vi "UHR-Fleezers Control (host) - 12.4.vi"() -> ()   [LabVIEW 2012] (continued)
  T20 = enum16{"empty", "write", "read oldest (queue)", "read newest (stack)", "read all"}
  T21 = cluster{"New Image":T2, "New Image":T2, "New Image":T2, "New Image":T2, "New Image":T2}
  T22 = typedef "XDNodeRunTimeDep.lvlib/timing_clust.ctl" = cluster{"Expected End [f-1]":u64, "Actual End [f-1]":u64, "Finished Late? [f-1]":bool, "Expected End [i-1]":u64, "Actual End [i-1]":u64, "Finished Late? [i-1]":bool, "Expected Start [i]":u64, "Actual Start [i]":u64, "Expected Start [f]":u64, "Actual Start [f]":u64, "Source Name":string, "Structure Name":string, "Period":i64, "Deadline":i64, "Offset":i64, "Start":i64, "Priority":i32, "Timeout":i32, "Mode":T23, "Wakeup Reason":T24, "Error":errorcluster, "Source Type":string, "Secondary Source Type":string, "Global End Time":u64, "Global Start Time":u64, "Frame Duration":u64, "Iteration Duration":u64, "Assigned CPU":i32, "I/O Scan Engine Mode":u32}
  T23 = typedef "XDNodeRunTimeDep.lvlib/nitl_modes.ctl" = enum32{"No Change", "Process missed periods, maintain original phase", "Discard missed periods, maintain original phase", "Process missed periods, ignore original phase", "Discard missed periods, ignore original phase"}
  T24 = typedef "XDNodeRunTimeDep.lvlib/wakeup.ctl" = enum32{"Normal", "Aborted", "Asynchronous wakeup", "Timing source error", "Timed loop error", "Timeout"}
  T25 = enum32{"Status", "Sample Stage", "Syringe Pump", "Trap Control (RF)", "APD Counting", "Fluorescence Laser Control", "Trap AI", "Video", "FPGA"}
  T26 = enum16{"big-endian, network order", "native, host order", "little-endian"}
  T27 = enum16{"open", "replace", "create", "open or create", "replace or create", "replace or create with confirmation"}
  T28 = cluster{"Scan Range AOD (nm) 2":dbl, "Step Size AOD (nm) 2":dbl, "Scan Speed AOD (nm/s) 2":dbl, "Number of scans (AOD) 2":u16, "Label":string}
  T29 = cluster{"[0]":dbl, "[1]":dbl, "[2]":dbl, "[3]":dbl, "[4]":dbl, "[5]":dbl}
  T30 = cluster{"Diameter (mm)":dbl, "Units":dbl, "Volume":dbl, "Rate":dbl}
  T31 = cluster{"Left":i32, "Top":i32, "Width":u32, "Height":u32}
  T32 = cluster{cluster{"Left":i32, "Top":i32, "Width":u32, "Height":u32}}[]
  T33 = enum32{"Normal Display", "Dual Display (APD)", "FFT", "High Res Display"}
  T34 = cluster{"Origin Pixel":cluster{"X":sgl, "Y":sgl}, "Angle Relative to Horizontal (deg)":sgl, "Axis Reference":u32}
  T35 = typedef "Simple Grid Descriptor" = cluster{"X Step":sgl, "Y Step":sgl, "Unit":T36}
  T36 = typedef "Image Unit" = enum32{"Undefined", "Angström", "Micrometer", "Millimeter", "Centimeter", "Meter", "Kilometer", "Microinch", "Inch", "Feet", "Nautical miles", "Standard miles", "Steps"}
  T37 = cluster{"averaging mode":u16, "weighting mode":u16, "number of averages":u32}
  T38 = cluster{"dB On (F)":bool, "unwrap phase (F)":bool, "convert to degree (F)":bool}
  T39 = cluster{string, string, string, string, string, string, string, string}
  T40 = cluster{string, string, string, string, string, string, string, string, string, string, string, string}
  T41 = cluster{string, string, string, string, string, string, string, string, string, string, string, string, string}
  T42 = cluster{string, string, string, string, string, string, string, string, string, string, string, string, string, string}
  T43 = cluster{"BD 1 Frequency 1 (MHz)":dbl, "BD 1 Frequency 2 (MHz)":dbl}
  T44 = cluster{"f0":dbl, "df":dbl, "magnitude":dbl[]}[][]
  T45 = enum32{"setting", "request", "request control", "info", "statistics", "system settings", "I/O sub system", "HRT control", "camera descriptions", "device specific data", "event sub system settings", "event sub system results", "image memory manager"}
  T46 = typedef "AviRefnum.ctl" = refnum<k1>
  T47 = typedef "imagedata.ctl" = cluster{"image type":i32, "image depth":i32, "image":u8[], "mask":u8[], "colors":u32[], "Rectangle":cluster{"left":i16, "top":i16, "right":i16, "bottom":i16}}
diagram:
  w3 = u16 10 items=["1.0"=10, "1.5"=15, "2.0"=20] ("stop bits (10: 1 bit)")
  w74 = u16 20 items=["1.0"=10, "1.5"=15, "2.0"=20] ("stop bits (10: 1 bit)")
  w77 = u16 20 items=["1.0"=10, "1.5"=15, "2.0"=20] ("stop bits (10: 1 bit)")
  w103 = u16 20 items=["1.0"=10, "1.5"=15, "2.0"=20] ("stop bits (10: 1 bit)")
  w9 = T17 2 items=["Grayscale (U8)", "Grayscale (I16)", "Grayscale (SGL)", "Complex (CSG)", "RGB (U32)", "HSL (U32)", "RGB (U64)", "Grayscale (U16)"] ("Image Type")
  w233 = 10.0 ("y")
  w232 = 32767.0 ("y")
  w248 = 6.0  # clock mult.
  w249 = 49152000.0  # TCXO frequ.
  # "What are these?"
  # "I don't think you need to do this.\nEverytime you want to adjust phase you always set this anyway.\nSince we removed the separate +/- controls.\n\nHaven't added for added fl lasers.  Should remove this code."
  # "Bottom 1 Harvard"
  # "Top 3 Harvard"
  # "Center Harvard"
  # "Bottom 1 Harvard"
  # "Top 3 Harvard"
  # "Center Harvard"
  n1 = Build Array("DIO count 1 (ticks)", "DIO count 2 (ticks)", "DIO count 3 (ticks)") -> (w154:u16[])
  n2 = xnode "Open FPGA VI Reference"("resource name"=T18 "750kHzDAQ") -> ("FPGA VI Reference Out"=w257:T19, "error out"=w256:errorcluster)  [unwired: 1 in]
  n3 = local read "AO1"() -> (w227:dbl)
  n4 = local read "AO2"() -> (w226:dbl)
  n5 = local read "Scan Increment (MHz)"() -> (w244:dbl)
  n6 = local read "Continuous MCL Scanning"() -> (w214:bool)
  n7 = local read "Fast Scan Dir"() -> (w213:bool)
  n8 = xnode "Invoke Method"("FPGA VI Reference In"=w257, "error in"=w256) -> ("FPGA VI Reference Out"=w13:T19, "error out"=w173:errorcluster)
  n9 = local read "Number of scans (MCL)"() -> (w215:u64)
  n10 = Multiply(x=w227, y=w232) -> (x*y=w229:dbl)
  n11 = Multiply(x=w226, y=w232) -> (x*y=w231:dbl)
  n12 = Divide(x=w229, y=w233) -> (x/y=w228:dbl)
  n13 = Divide(x=w231, y=w233) -> (x/y=w230:dbl)
  n14 = To Word Integer(number=w228) -> (16bit integer=w225:i16)
  n15 = To Word Integer(number=w230) -> (16bit integer=w224:i16)
  n16 = Not(x=w213) -> (.not. x?=w208:bool)
  n17 = local read "Cycles/step (MCL)"() -> (w216:u64)
  n18 = Multiply(x=w244, y=1000.0) -> (x*y=w251:dbl)
  n19 = local read "Scan steps (MCL)"() -> (w217:u64)
  n20 = local read "Desired Scan Incr (V)"() -> (w219:dbl)
  n21 = Scale By Power Of 2(n=48, x=w251) -> (x*2^n=w252:dbl)
  n22 = Unbundle By Name(cluster{"output high":i16, "output low":i16} {"output high"=3000, "output low"=0} ("FB output range 1")) -> ("output high"=w55:i16, "output low"=w54:i16)
  n23 = Multiply(x=w249, y=w248) -> (x*y=w247:dbl)
  n24 = Divide(x=w252, y=w247) -> (x/y=w246:dbl)
  n25 = local read "Setpoints (V)"() -> (w263:cluster{"Set 1":dbl, "Set 2":dbl})
  n26 = To Quad Integer(1:w246) -> (0:w243:i64)
  n27 = Divide(x=40000000.0, y="AI Count (ticks)") -> (x/y=w204:dbl)
  n28 = Multiply(x=w219, y=32767.0) -> (x*y=w221:dbl)
  n29 = local read "Trap Intensity PID Gains"() -> (w258:T9)
  n30 = local write "Trap Pos FIFO Timeout"(u16 0 ("Trap Pos FIFO Timeout")) -> ()
  n31 = local read "Number Interlace Sets"() -> (w147:u8)
  n32 = Split 1D Array(array=w154, index=w147) -> (first subarray=w156:u16[])  [unwired: 1 out]
  n33 = Add Array Elements(numeric array=w156) -> (sum=w155:u16)
  n34 = local read "# Samples/channel"() -> (w236:u32)
  n35 = local read "Number of F/B Scans (AOD)"() -> (w237:u16)
  n36 = local read "Not-Interlacing Set"() -> (w146:enum32{"Set 1", "Set 2", "Set 3"})
  n37 = To Unsigned Byte Integer(number=w146) -> (unsigned 8bit integer=w152:u8)
  n38 = Index Array(array=w154, index=w152) -> (element=w153:u16)
  n39 = local read "Feedback On/Off"() -> (w266:cluster{"Set 1":bool, "Set 2":bool})
  n40 = local read "Scan steps (AOD)"() -> (w242:u64)
  n41 = local read "All FB On/Off"() -> (w267:bool)
  n42 = local read "Cycles/step (AOD)"() -> (w241:u64)
  n43 = local write "AI rate (Hz)"(w204) -> ()
  n44 = Divide(x=w221, y=10.0) -> (x/y=w220:dbl)
  n45 = Multiply(x=w242, y=w241) -> (x*y=w240:u64)
  n46 = Unbundle By Name(w258) -> ("proportional gain (Kc)"=w59:i16, "integral gain (Kc*Ts/Ti)"=w58:i16, "derivative gain (Kc*Td/Ts)"=w57:i16)
  n47 = property on="AI Count (ticks)" class="DigNum (strict)"("Val(Sgnl)"="AI Count (ticks)") -> ()  [unwired: 2 in, 2 out]
  n48 = Multiply(x=3276.7, y=w263) -> (x*y=w262:cluster{"Set 1":dbl, "Set 2":dbl})
  n49 = To Word Integer(number=w220) -> (16bit integer=w218:i16)
  n50 = Multiply(x=w240, y=u64 2) -> (x*y=w238:u64)
  n51 = Divide(x=w204, y="FPGA Ave.") -> (x/y=w205:dbl)
  n52 = To Word Integer(number=w262) -> (16bit integer=w261:cluster{"Set 1":i16, "Set 2":i16})
  n53 = Multiply(x=w238, y=w237) -> (x*y=w235:u64)
  n54 = local read "Sets to FIFO (Traps)"() -> (w63:T15)
  n55 = local write "Ave. Rate (Hz)"(w205) -> ()
  n56 = Divide(x=w235, y=w236) -> (x/y=w234:dbl)
  n57 = Unbundle By Name(w261) -> ("Set 1"=w260:i16, "Set 2"=w259:i16)
  n58 = local read "2D or 1D Scan"() -> (w165:bool)
  n59 = local write "Data points/scans"(w235) -> ()
  n60 = local read "Scan BD"() -> (w253:bool)
  n61 = And(x=w266, y=w267) -> (x .and. y?=w265:cluster{"Set 1":bool, "Set 2":bool})
  n62 = local write "Data points/scan (f/b)"(w238) -> ()
  n63 = Reciprocal(x=w205) -> (1/x=w206:dbl)
  n64 = local read "N Acq Sets (Traps + Fl.)"() -> (w197:i16)
  n65 = local write "N sets should be saved"(w234) -> ()
  n66 = Unbundle By Name(w265) -> ("Set 1"=w269:bool, "Set 2"=w268:bool)
  n67 = local read "Interlace"() -> (w148:bool)
  n68 = Select(t=w155, s=w148, f=w153) -> (s? t:f=w145:u16)
  n69 = local write "Update Count (MCL)"(w145) -> ()
  n70 = local write "Total Counts (ticks)"(w145) -> ()
  n71 = local write "Ave. Period (s)"(w206) -> ()
  n72 = Unbundle By Name(w63) -> ("Set 1"=w62:bool, "Set 2"=w61:bool, "Set 3"=w60:bool)
  n73 = property on="2D or 1D Scan" class="Bool (strict)"("Val(Sgnl)"=w165) -> ()  [unwired: 2 in, 2 out]
  n74 = xnode "Read/Write Control"("FPGA VI Reference In"=w164, "error in"=w173, "ai count"="AI Count (ticks)", "Interlace ON/OFF"=w148, "Number Interlace Cycles"=w147, "Set 1"=w62, "Set 2"=w61, "Set 3"=w60, "FB On/Off Set 1"=w269, "FB On/Off Set 2"=w268, "Interlace Off Parameters"=w146, "FB Setpoint Set 1"=w260, "FB Setpoint Set 2"=w259, "P1"=w59, "I1"=w58, "D1"=w57, "FB1 output high"=w55, "FB1 output low"=w54, "Cycles per step"=w241, "Scan BD"=w253, "Number of scans"=w237, "Scan steps"=w242, "Scan freq.  increment"=w243, "AO1"=w225, "AO2"=w224, "Scan freq.  increment (MCL)"=w218, "Scan steps (MCL)"=w217, "Cycles per step (MCL)"=w216, "Number of scans (MCL)"=w215, "MCL count"=w145, "Cont. Scan (MCL)"=w214, "MCL Scan Axis"=w208, "1D or 2D Scan?"=w165, "N of AI1 Int Acq Sets"=w197, "Amp switch delay"="Amp switch delay", "Swap F1 and F2"="Swap F1 and F2", "APD to FIFO"=FALSE, "DIO count 1 (ticks)"="DIO count 1 (ticks)", "DIO count 2 (ticks)"="DIO count 2 (ticks)", "DIO count 3 (ticks)"="DIO count 3 (ticks)") -> ("FPGA VI Reference Out"=w15:T19, "error out"=w14:errorcluster)  [unwired: 1 in]
  n75 = local read "Laser interlacing mode"() -> (w144:enum32{"Laser ON", "Laser OFF", "Interlace"})
  n76 = local read "Green Laser ON"() -> (w143:bool)
  n77 = local read "Trap Pos. FB Range"() -> (w53:T12)
  n78 = local read "Trap Pos. FB Gains"() -> (w52:T11)
  n79 = Multiply(x="Green Intensity % (FB OFF)", y=655.35) -> (x*y=w136:dbl)
  n80 = local read "Invert laser interlacing"() -> (w30:bool)
  n81 = local read "Trap Pos. AI1 X Pre-scale"() -> (w91:u16)
  n82 = Multiply(x="Green FB Setpoint (mV)", y=3.2767) -> (x*y=w133:dbl)
  n83 = local read "Trap Pos FB Int Count"() -> (w85:u16)
  n84 = local read "Differential FB?"() -> (w79:bool)
  n85 = local read "Neg. TTrig FPGA"() -> (w81:bool)
  n86 = Multiply(x="Red FB Setpoint (mV)", y=3.2767) -> (x*y=w39:dbl)
  n87 = To Unsigned Word Integer(number=w136) -> (unsigned 16bit integer=w134:u16)
  n88 = Multiply(x="Red Intensity % (FB OFF)", y=655.35) -> (x*y=w35:dbl)
  n89 = To Word Integer(number=w133) -> (16bit integer=w131:i16)
  n90 = Unbundle By Name("Green FB Gains") -> ("proportional gain (Kc)"=w44:i16, "integral gain (Kc*Ts/Ti)"=w43:i16, "derivative gain (Kc*Td/Ts)"=w42:i16)
  n91 = case shown="False" w143 {
    tunnel: w144 -> [_ w295]
    tunnel: [enum32{"Laser ON", "Laser OFF", "Interlace"}."Laser OFF" ("Green laser mode") w295] -> w29
    frame False {
    }
    frame True {
    }
  }
  n92 = To Word Integer(number=w39) -> (16bit integer=w36:i16)
  n93 = Unbundle By Name("Red FB Gains") -> ("proportional gain (Kc)"=w27:i16, "integral gain (Kc*Ts/Ti)"=w26:i16, "derivative gain (Kc*Td/Ts)"=w25:i16)
  n94 = Unbundle By Name(w52) -> ("proportional gain (Kc)"=w48:fxp<+/-,16,8>, "integral gain (Kc*Ts/Ti)"=w47:fxp<+/-,16,8>, "derivative gain (Kc*Td/Ts)"=w46:fxp<+/-,16,8>)
  n95 = To Unsigned Word Integer(number=w35) -> (unsigned 16bit integer=w32:u16)
  n96 = Unbundle By Name(w53) -> ("output high"=w51:fxp<+/-,16,1>, "output low"=w49:fxp<+/-,16,1>)
  n97 = local read "Trap Pos FB Monitor\nT1 or T2"() -> (w96:bool)
  n98 = local read "Trap Pos FB Negate Action"() -> (w95:bool)
  n99 = local read "Trap Pos. FB Offset Factor"() -> (w94:i64)
  n100 = local read "Trap Pos. FB Mult Factor"() -> (w93:i64)
  n101 = xnode "Read/Write Control"("FPGA VI Reference In"=w15, "error in"=w14, "Invert GI 2"=w30, "Operating Mode 2"=w29, "P3"=w44, "I3"=w43, "D3"=w42, "Green FB Setpoint"=w131, "Green FB On/Off"="Green FB On/Off", "Current Out"=w134, "Green int current ON count adj"="Green int current ON count adj", "Operating Mode"=w29, "Invert GI"=w30, "Trap Pos FB Monitor T1 or T2"=w96, "Trap Pos FB Negate Action"=w95, "Trap Pos. FB Offset Factor"=w94, "Trap Pos. FB Mult Factor"=w93, "Force feedback"=FALSE, "AI1 X Scale"=w91, "Trap Pos to FIFO"=TRUE, "Trap Pos FB Int Count"=w85, "TTrig Negate Pos"=w81, "FB Trig Integrate"="FB Trig Integrate", "Diff FB Measurement?"=w79, "Negate Diff?"="Negate Diff?", "P2"=w48, "I2"=w47, "D2"=w46, "FB2 output high"=w51, "FB2 output low"=w49, "Red FB Setpoint"=w36, "RI Current Out"=w32, "Red int current ON count adj"="Red int current ON count adj", "Red Laser Operating Mode"=w29, "RI Operating Mode 2"=w29, "Invert RI 2"=w30, "Invert RI"=w30, "P4"=w27, "I4"=w26, "D4"=w25, "Red FB On/Off"="Red FB On/Off") -> ("FPGA VI Reference Out"=w20:T19, "error out"=w22:errorcluster)
  n102 = stacked-sequence {
    tunnel: w22 -> [_ _ w304]
    tunnel: [_ _ w304] -> w21
    tunnel: w20 -> [_ _ w305]
    tunnel: [_ _ w305] -> w19
    frame #0 {
      w296 = T20."empty" ("mode")
      # "Clear external fluorescence triggering FIFO"
      # "APD loop counts"
      # "Fluorescence loop counts (rates)"
      n103 = local read "APD Integration Time (s)"() -> (w298:dbl)
      n104 = local read "Interlace ON count"() -> (w299:u16)
      n105 = call "Smart Buffer (DBL) 1.vi"("mode"=w296) -> ()  [unwired: 5 in, 6 out]
      n106 = call "Smart Buffer (DBL) 2.vi"("mode"=w296) -> ()  [unwired: 5 in, 6 out]
      n107 = property on="APD Integration Time (s)" class="DigNum (strict)"("Val(Sgnl)"=w298) -> ()  [unwired: 2 in, 2 out]
      n108 = property on="Interlace ON count" class="DigNum (strict)"("Val(Sgnl)"=w299) -> ()  [unwired: 2 in, 2 out]
      "Number of APDs" <- 3.0 ("Number of APDs")
    }
    frame #1 {
      # "Number of APDs affects\nAPD DMA transfer"
      # "General settings for all lasers:"
      # "And includes all laser\nON/OFF settings"
      # "Fluorescent lasers settings:"
      # "Blue laser settings:"
      n109 = local read "Laser interlacing mode"() -> (w301:enum32{"Laser ON", "Laser OFF", "Interlace"})
      n110 = local read "Invert laser interlacing"() -> (w300:bool)
      n111 = local read "Blue FB On/Off"() -> (w302:bool)
      n112 = property on="Blue FB On/Off" class="Bool (strict)"("Val(Sgnl)"=w302) -> ()  [unwired: 2 in, 2 out]
      n113 = property on="Invert laser interlacing" class="Bool (strict)"("Val(Sgnl)"=w300) -> ()  [unwired: 2 in, 2 out]
      n114 = property on="Laser interlacing mode" class="RadioBtnsControl (strict)"("Val(Sgnl)"=w301) -> ()  [unwired: 2 in, 2 out]
    }
    frame #2 {
      n115 = Wait (ms)(milliseconds to wait=u32 1000) -> ()  [unwired: 1 out]
    }
  }
  n116 = local write "Offset (nm)"(0.0 ("Offset (nm)")) -> ()
  n117 = local write "Bead Mean (nm)"(0.0 ("Bead Mean (nm)")) -> ()
  n118 = xnode "Invoke Method"("FPGA VI Reference In"=w19, "error in"=w21, "Requested Depth"="Trap AI FIFO Depth") -> ("FPGA VI Reference Out"=w99:T19, "error out"=w98:errorcluster)  [unwired: 1 out]
  n119 = xnode "Invoke Method"("FPGA VI Reference In"=w99, "error in"=w98, "Requested Depth"="Trap Position FIFO Depth") -> ("FPGA VI Reference Out"=w87:T19, "error out"=w86:errorcluster)  [unwired: 1 out]
  n120 = flat-sequence "Safety limits on RF frequencies and amplitudes (for AOM protection)" {
    tunnel: w13 -> [w310]
    tunnel: [w310] -> w164
    tunnel: [w309] -> w163
    tunnel: [w308] -> w162
    tunnel: [w306] -> w160
    tunnel: [w307] -> w161
    frame #0 {
      w307 = T16 {"Minimum"=0.0, "Maximum"=40.0, "Increment"=1.0} ("Min Max Inc")
      w306 = T16 {"Minimum"=0.0, "Maximum"=50.0, "Increment"=1.0} ("Data Entry Limits")
      w309 = T16 {"Minimum"=60.0, "Maximum"=90.0, "Increment"=1.0} ("Min Max Inc")
      w308 = T16 {"Minimum"=0.0, "Maximum"=50.0, "Increment"=1.0} ("Data Entry Limits")
      n121 = property on="BD 2 Frequency 1 (MHz)" class="DigNum (strict)"("Data Range"=w307) -> ()  [unwired: 2 in, 2 out]
      n122 = property on="BD 2 Frequency 3 (MHz)" class="DigNum (strict)"("Data Range"=w307) -> ()  [unwired: 2 in, 2 out]
      n123 = property on="BD 2 Frequency 2 (MHz)" class="DigNum (strict)"("Data Range"=w307) -> ()  [unwired: 2 in, 2 out]
      n124 = property on="BD 1 Frequency 1 (MHz)" class="DigNum (strict)"("Data Range"=w309) -> ()  [unwired: 2 in, 2 out]
      n125 = property on="BD 1 Frequency 2 (MHz)" class="DigNum (strict)"("Data Range"=w309) -> ()  [unwired: 2 in, 2 out]
      n126 = property on="BD 1 Frequency 3 (MHz)" class="DigNum (strict)"("Data Range"=w309) -> ()  [unwired: 2 in, 2 out]
      n127 = property on="BD 2 Amplitude 1 (%)" class="DigNum (strict)"("Data Range"=w306) -> ()  [unwired: 2 in, 2 out]
      n128 = property on="BD 2 Amplitude 2 (%)" class="DigNum (strict)"("Data Range"=w306) -> ()  [unwired: 2 in, 2 out]
      n129 = property on="BD 2 Amplitude 3 (%)" class="DigNum (strict)"("Data Range"=w306) -> ()  [unwired: 2 in, 2 out]
      n130 = property on="BD 1 Amplitude 3 (%)" class="DigNum (strict)"("Data Range"=w308) -> ()  [unwired: 2 in, 2 out]
      n131 = property on="BD 1 Amplitude 2 (%)" class="DigNum (strict)"("Data Range"=w308) -> ()  [unwired: 2 in, 2 out]
      n132 = property on="BD 1 Amplitude 1 (%)" class="DigNum (strict)"("Data Range"=w308) -> ()  [unwired: 2 in, 2 out]
      "X RF Frequency Limits (MHz)" <- w309
      "X RF Amplitude Limits (%)" <- w308
      "Y RF Amplitude Limits (%)" <- w306
      "Y RF Frequency Limits (MHz)" <- w307
    }
  }
  n133 = xnode "Invoke Method"("FPGA VI Reference In"=w87, "error in"=w86) -> ("FPGA VI Reference Out"=w172:T19, "error out"=w171:errorcluster)  [unwired: 1 in]
  n134 = flat-sequence "Initial FPGA Loop Relative Phase Adjustment" {
    tunnel: "Initial Phase Adjustment (AI1)" -> [w328]
    tunnel: "Initial Phase Adjustment (GI)" -> [w327]
    tunnel: w172 -> [w326]
    tunnel: w171 -> [w325]
    tunnel: "Initial Phase Adj. (MCL)" -> [w324]
    tunnel: [w329] -> w181
    tunnel: [w323] -> w177
    tunnel: "Initial Phase Adjustment (APD Acq)" -> [w322]
    tunnel: "Initial Phase Adjustment (APD 1 Gate)" -> [w321]
    tunnel: "Initial Phase Adjustment (Green FB)" -> [w320]
    tunnel: "Initial Phase Adjustment (GI) 2" -> [w319]
    tunnel: "Initial Phase Adjustment (APD 2 Gate)" -> [w318]
    tunnel: "Initial Phase Adjustment (RI)" -> [w317]
    tunnel: "Initial Phase Adjustment (RI) 2" -> [w316]
    tunnel: "Initial Phase Adjustment (RI FB)" -> [w315]
    tunnel: "Initial Phase Adjustment (BI DO)" -> [w314]
    tunnel: "Initial Phase Adjustment (BI AO)" -> [w313]
    tunnel: "Initial Phase Adjustment (BI AI)" -> [w312]
    tunnel: "Initial Phase Adjustment (APD 3 Gate)" -> [w311]
    tunnel: w181 -> [w331]
    tunnel: [w332] -> w178
    tunnel: w177 -> [w332]
    tunnel: [w331] -> w176
    tunnel: w178 -> [w335]
    tunnel: w176 -> [w334]
    tunnel: [w337] -> w175
    tunnel: [w336] -> w174
    tunnel: [w339] -> w179
    tunnel: [w340] -> w180
    tunnel: w175 -> [w340]
    tunnel: w174 -> [w339]
    frame #0 {
      n135 = xnode "Read/Write Control"("FPGA VI Reference In"=w326, "error in"=w325, "Phase count adjustment"=w328, "Phase count adjustment (GI)"=w327, "Phase count adjustment (MCL)"=w324, "Phase Count Adjustment (APD Acq)"=w322, "Phase count adjustment (APD 1 Gate)"=w321, "Phase count adjustment (APD 2 Gate)"=w318, "Phase count adjustment (Green FB)"=w320, "Phase count adjustment (GI) 2"=w319, "Phase count adjustment (RI)"=w317, "Phase count adjustment (RI) 2"=w316, "Phase count adjustment (Red FB)"=w315, "Phase count adjustment (BI AO)"=w313, "Phase count adjustment (BI D)"=w314, "Phase count adjustment (Blue Int)"=w312, "Phase count adjustment (APD 3 Gate)"=w311) -> ("FPGA VI Reference Out"=w323:T19, "error out"=w329:errorcluster)
    }
    frame #1 {
      n136 = Wait (ms)(milliseconds to wait=u32 100) -> ()  [unwired: 1 out]
    }
    frame #2 {
      w333 = TRUE
      n137 = xnode "Read/Write Control"("FPGA VI Reference In"=w335, "error in"=w334, "+ phase"=w333, "+ phase (GI)"=w333, "+ phase (MCL)"=w333, "+ phase (APD Acq)"=w333, "+ phase (APD 1 Gate)"=w333, "+ phase (APD 2 Gate)"=w333, "+ phase (Green FB)"=w333, "+ phase (GI) 2"=w333, "+ phase (RI)"=w333, "+ phase (RI) 2"=w333, "+ phase (BI AO)"=w333, "+ phase (BI D)"=w333, "+ phase (Blue Int)"=w333, "+ phase (APD 3 Gate)"=w333) -> ("FPGA VI Reference Out"=w336:T19, "error out"=w337:errorcluster)
    }
    frame #3 {
      n138 = Wait (ms)(milliseconds to wait=u32 100) -> ()  [unwired: 1 out]
    }
  }
  n139 = local read "Phase adj. (Green FB)"() -> (w157:i16)
  n140 = local read "Phase adj. (GI) 2"() -> (w137:i16)
  n141 = local read "Phase adjust (MCL)"() -> (w209:i16)
  n142 = local read "Phase adj. (AI1)"() -> (w211:i16)
  n143 = local read "Phase adj. (GI)"() -> (w210:i16)
  n144 = xnode "Read/Write Control"("FPGA VI Reference In"=w179, "error in"=w180, "Phase count adjustment"=w211, "Phase count adjustment (GI)"=w210, "Phase count adjustment (MCL)"=w209, "Phase Count Adjustment (APD Acq)"="Phase Adj. (APD Acq)", "Phase count adjustment (APD 1 Gate)"="Phase Adj. (APD 1 Gate)", "Phase count adjustment (APD 2 Gate)"="Phase Adj. (APD 2 Gate)", "Phase count adjustment (Green FB)"=w157, "Phase count adjustment (GI) 2"=w137) -> ("FPGA VI Reference Out"=w123:T19, "error out"=w186:errorcluster)
  n145 = call "Initialize RF boards - interlace 3.vi"("error in"=w186, "FPGA VI Reference In"=w123) -> ("error out"=w184:errorcluster, "FPGA VI Reference Out"=w185:T19)
  n146 = call "set RF board frequency - interlace.vi"("Board 2 Frequency Limits"=w161, "Board 1 Frequency Limits"=w163, "error in"=w184, "FPGA VI Reference In"=w185, "Board 2 Frequency 3 (MHz)"="BD 2 Frequency 3 (MHz)", "Board 1 Frequency 3 (MHz)"="BD 1 Frequency 3 (MHz)", "Board 2 Frequency 2 (MHz)"="BD 2 Frequency 2 (MHz)", "Board 2 Frequency 1 (MHz)"="BD 2 Frequency 1 (MHz)", "Board 1 Frequency 2 (MHz)"="BD 1 Frequency 2 (MHz)", "Board 1 Frequency 1  (MHz)"="BD 1 Frequency 1 (MHz)") -> ("error out"=w284:errorcluster, "FPGA VI Reference Out"=w285:T19)
  n147 = call "set RF board amplitude - interlace.vi"("Board 2 Amplitude Limits"=w160, "Board 1 Amplitude Limits"=w162, "error in"=w284, "FPGA VI Reference In"=w285, "Board 2 Amplitude 3 (%)"="BD 2 Amplitude 3 (%)", "Board 1 Amplitude 3 (%)"="BD 1 Amplitude 3 (%)", "Board 2 Amplitude 2 (%)"="BD 2 Amplitude 2 (%)", "Board 2 Amplitude 1 (%)"="BD 2 Amplitude 1 (%)", "Board 1 Amplitude 2 (%)"="BD 1 Amplitude 2 (%)", "Board 1 Amplitude 1 (%)"="BD 1 Amplitude 1 (%)") -> ("error out"=w272:errorcluster, "FPGA VI Reference Out"=w273:T19)
  n148 = flat-sequence {
    tunnel: w273 -> [w350]
    tunnel: w272 -> [w349]
    tunnel: [w348] -> w277
    tunnel: [w347] -> w276
    tunnel: [w354] -> w275
    tunnel: w277 -> [w354]
    tunnel: [w353] -> w274
    tunnel: w276 -> [w353]
    tunnel: w275 -> [w363]
    tunnel: w274 -> [w362]
    tunnel: [w361] -> w12
    tunnel: [w360] -> w88
    frame #0 {
      w341 = FALSE ("Retract Pump 3")
      n149 = local read "Trap 1 (ON/OFF)"() -> (w342:bool)
      n150 = xnode "Read/Write Control"("FPGA VI Reference In"=w350, "error in"=w349, "Direct RF Box  Communication"=FALSE) -> ("FPGA VI Reference Out"=w348:T19, "error out"=w347:errorcluster)
      n151 = local write "Saving..."(FALSE ("Saving Data")) -> ()
      n152 = local write "Stop All"(FALSE ("Stop All")) -> ()
      n153 = local write "Retract Pump 1"(w341) -> ()
      n154 = local write "Retract Pump 3"(w341) -> ()
      n155 = local write "Index"(1.0 ("Index")) -> ()
      n156 = property on="Trap 1 ON" class="Bool (strict)"("Value"=w342) -> ()  [unwired: 2 in, 2 out]
      "Manipulating Trap" <- FALSE ("Manipulating Trap")
    }
    frame #1 {
      n157 = local read "Trap 2 (ON/OFF)"() -> (w352:bool)
      n158 = Wait (ms)(milliseconds to wait=u32 10) -> ()  [unwired: 1 out]
      n159 = property on="Trap 2 ON" class="Bool (strict)"("Val(Sgnl)"=w352) -> ()  [unwired: 2 in, 2 out]
    }
    frame #2 {
      n160 = local read "Scan Range (nm)"() -> (w356:dbl)
      n161 = xnode "Read/Write Control"("FPGA VI Reference In"=w363, "error in"=w362, "FPGA Controls  RF Box"=TRUE ("Direct RF Box  Communication")) -> ("FPGA VI Reference Out"=w361:T19, "error out"=w360:errorcluster)
      n162 = call "Update messages.vi"("Message to add"="UHR-Fleezers ready.", "Old message string"="") -> ("New message string"=w359:string)
      n163 = local write "Messages"(w359) -> ()
      n164 = property on="Scan Range (nm)" class="DigNum (strict)"("Val(Sgnl)"=w356) -> ()  [unwired: 2 in, 2 out]
    }
  }
  n165 = Subtract(x="BD 1 Frequency 1 (MHz)", y="BD 1 Frequency 2 (MHz)") -> (x-y=w196:dbl)
  n166 = Subtract(x="BD 2 Frequency 1 (MHz)", y="BD 2 Frequency 2 (MHz)") -> (x-y=w195:dbl)
  n167 = Square(x=w195) -> (x^2=w193:dbl)
  n168 = Square(x=w196) -> (x^2=w194:dbl)
  n169 = Add(x=w194, y=w193) -> (x+y=w192:dbl)
  n170 = Square Root(x=w192) -> (sqrt(x)=w191:dbl)
  n171 = local write "Trap Delta (MHz)"(w191) -> ()
  n172 = call-poly "VISA Configure Serial Port"("VISA resource name"="VISA resource name", "baud rate (9600)"=u32 115200, "stop bits (10: 1 bit)"=w3) -> ("VISA resource name out"=w2:refnum<visa-resource-name>, "error out"=w1:errorcluster)  [unwired: 4 in, 7 out]
  n173 = call-poly "VISA Configure Serial Port"("VISA resource name"="Bottom  1 Harvard Syringe Pump Serial Port", "baud rate (9600)"=u32 115200, "stop bits (10: 1 bit)"=w74) -> ("VISA resource name out"=w70:refnum<visa-resource-name>, "error out"=w69:errorcluster)  [unwired: 4 in, 7 out]
  n174 = call-poly "VISA Configure Serial Port"("VISA resource name"="Top 3 Harvard Syringe Pump Serial Port", "baud rate (9600)"=u32 115200, "stop bits (10: 1 bit)"=w77) -> ("VISA resource name out"=w72:refnum<visa-resource-name>, "error out"=w71:errorcluster)  [unwired: 4 in, 7 out]
  n175 = call-poly "VISA Configure Serial Port"("VISA resource name"="Sample Chamber Stage Serial Port") -> ("VISA resource name out"=w118:refnum<visa-resource-name>, "error out"=w119:errorcluster)  [unwired: 5 in, 8 out]
  "Stage Control Serial Error" <- w119
  n176 = local write "Blue Error Out"(w1) -> ()
  n177 = call-poly "VISA Configure Serial Port"("VISA resource name"="Center Harvard Syringe Pump Serial Port", "baud rate (9600)"=u32 115200, "stop bits (10: 1 bit)"=w103) -> ("VISA resource name out"=w100:refnum<visa-resource-name>, "error out"=w101:errorcluster)  [unwired: 4 in, 7 out]
  n178 = call "IMAQ Create"("Image Name"="APD 1 Image", "Image Type"=w9) -> ("New Image"=w109:T2)  [unwired: 3 in, 1 out]
  n179 = call "IMAQ Create"("Image Name"="APD 2 Image", "Image Type"=w9) -> ("New Image"=w108:T2)  [unwired: 3 in, 1 out]
  n180 = call "IMAQ Create"("Image Name"="APD 3 Image", "Image Type"=w9) -> ("New Image"=w8:T2)  [unwired: 3 in, 1 out]
  n181 = call "IMAQ Create"("Image Name"="Det. X Image", "Image Type"=w9) -> ("New Image"=w107:T2)  [unwired: 3 in, 1 out]
  n182 = call "IMAQ Create"("Image Name"="Det. Y Image", "Image Type"=w9) -> ("New Image"=w106:T2)  [unwired: 3 in, 1 out]
  n183 = Bundle("New Image"=w109, "New Image"=w108, "New Image"=w8, "New Image"=w107, "New Image"=w106) -> (w105:T21)  [unwired: 1 in]
  n184 = node-c288(3 ("Processor")) -> (w125:T22)  [unwired: 3 out]
  n185 = node-c288() -> (w114:T22)  [unwired: 4 in]
  n186 = node-c288(2 ("Processor")) -> (w127:T22)  [unwired: 3 out]
  n187 = node-c288() -> (w129:T22)  [unwired: 4 out]
  n188 = node-c288(i64 1 ("Period"), 1 ("Processor")) -> (w200:T22)  [unwired: 2 out]
  n189 = node-c288() -> (w7:T22)  [unwired: 4 out]
  n190 = timed-loop "Oscillate Trap/AOM (fishing, conjugate plane alignment)" {
    tunnel: w13 -> [w366]
    tunnel: [w365] -> w130
    timing: w125 -> [_]
    timing-out: [_] -> w124
    stop <- w365 stop-if-true
    n191 = node-c288() -> ()  [unwired: 2 out]
    n192 = event shown="[1] \"Fl. Triggered...\": Value Change" {
      selector: _ -> [_ _ _]
      dyn-events: _ -> [_ _ _]
      timeout: _ -> [_ _ _]
      tunnel: w366 -> [w373 _ _]
      tunnel: [FALSE ("Stop All") _ w962] -> w365
      event "Oscillate Set 1", "Fish for Tether": Value Change {
        n193 = event-data() -> ()  [unwired: 6 out]
        n194 = local read "Oscillate Set 1"() -> (w372:bool)
        n195 = Or(x=w372, y="Fish for Tether") -> (x .or. y?=w370:bool)
        n196 = case shown="True" w370 {
          tunnel: w373 -> [_ w376]
          tunnel: "Fish for Tether" -> [_ w375]
          frame False {
          }
          frame True {
            n197 = case shown="True" w375 {
              selector: w375 -> [w379 w385]
              tunnel: [w379 w385] -> w374
              frame False {
              }
              frame True {
                n198 = local write "Scan axis 2"(TRUE) -> ()
                n199 = local write "Tether"(FALSE ("Tether")) -> ()
                n200 = local read "Flow ON during cal?"() -> (w380:bool)
                n201 = property on="Trap Delta (MHz)" class="DigNum (strict)"("Val(Sgnl)"="Furthest Delta (MHz)") -> ()  [unwired: 2 in, 2 out]
                n202 = Or(x="Flow ON during \nfishing?", y=w380) -> (x .or. y?=w381:bool)
                n203 = Wait (ms)(milliseconds to wait=u32 500) -> ()  [unwired: 1 out]
                n204 = property on="Sample Channel\nFlow" class="Bool (strict)"("Val(Sgnl)"=w381) -> ()  [unwired: 2 in, 2 out]
              }
            }
            n205 = node-c288() -> (w378:T22)  [unwired: 4 out]
            n206 = timed-loop "Oscillate AOD" {
              timing: w378 -> [_]
              timing-out: [_] -> w377
              tunnel: w376 -> [w395]
              tunnel: w374 -> [w388]
              i -> [w397]
              stop <- w394 stop-if-true
              n207 = node-c288() -> (w396:i64)  [unwired: 1 out]
              n208 = flat-sequence {
                tunnel: w397 -> [w424]
                tunnel: w396 -> [w423]
                tunnel: w395 -> [w402]
                tunnel: w388 -> [w405]
                tunnel: [w405] -> w393
                tunnel: [w404] -> w392
                tunnel: [w401] -> w391
                tunnel: [w398] -> w389
                tunnel: w393 -> [w460]
                tunnel: w392 -> [w458]
                tunnel: w391 -> [w457]
                tunnel: [w456] -> w390
                tunnel: w389 -> [w455]
                tunnel: [w532] -> w394
                tunnel: w390 -> [w531]
                frame #0 {
                  n209 = Divide(x=w423, y=i64 1000) -> (x/y=w418:dbl)
                  n210 = local read "BD 1 Frequency 2 (MHz)"() -> (w403:dbl)
                  n211 = Multiply(x="Osc. freq. (Hz)", y=6.283185307179586) -> (x*y=w421:dbl)
                  n212 = Multiply(x=w418, y=w424) -> (x*y=w420:dbl)
                  n213 = Multiply(x=w421, y=w420) -> (x*y=w400:dbl)
                  n214 = local read "BD 1 Frequency 1 (MHz)"() -> (w408:dbl)
                  n215 = local read "BD 2 Frequency 1 (MHz)"() -> (w407:dbl)
                  n216 = case shown="True" w405 {
                    tunnel: w400 -> [w430 w435]
                    tunnel: w408 -> [_ w446]
                    tunnel: w403 -> [_ w447]
                    tunnel: [w427 w441] -> w406
                    tunnel: [FALSE w438] -> w401
                    tunnel: [0.0 w431] -> w398
                    frame False {
                      n217 = Sine(x=w430) -> (sin(x)=w428:dbl)
                      n218 = Multiply(x=w428, y="Osc. amp. (MHz)") -> (x*y=w427:dbl)
                    }
                    frame True {
                      n219 = Cosine(x=w435) -> (cos(x)=w450:dbl)
                      n220 = Subtract(x=w447, y=w446) -> (x-y=w445:dbl)
                      n221 = Decrement(x=w450) -> (x-1=w449:dbl)
                      n222 = Subtract(x=w445, y="Closest Delta (MHz)") -> (x-y=w442:dbl)
                      n223 = Divide(x=w449, y=-2.0) -> (x/y=w443:dbl)
                      n224 = Multiply(x=w443, y=w442) -> (x*y=w441:dbl)
                      n225 = local read "Vec Mean of T1 T2"() -> (w437:dbl[])
                      n226 = Greater?(x=w437, y="Stop F (pN)") -> (0:w439:bool[])
                      n227 = Or Array Elements(Boolean array=w439) -> (logical OR=w438:bool)
                      n228 = Divide(x=w435, y=6.283185307179586) -> (x/y=w434:dbl)
                      n229 = Round Toward +Infinity(x=w434) -> (ceil(x): smallest int >= x=w431:dbl)
                      "Attempts" <- w431
                      n230 = Greater?(x=w431, y="Attempt Limit") -> (0:w433:bool)
                      n231 = case shown="True" w433 {
                        frame False {
                        }
                        frame True {
                          n232 = local write "Fish for Tether"(FALSE ("Fish for Tether")) -> ()
                          n233 = call <vilib>:"Beep.vi"() -> ()  [unwired: 3 in, 9 out]
                          n234 = local read "Messages"() -> (w452:string)
                          n235 = call "Update messages.vi"("Message to add"="Tether fishing timeout." ("Messages"), "Old message string"=w452) -> ("New message string"=→"Messages":string)
                        }
                      }
                    }
                  }
                  n236 = Select(t=w408, s="Scan axis 2", f=w407) -> (s? t:f=w411:dbl)
                  n237 = Add(x=w406, y=w411) -> (x+y=w404:dbl)
                  n238 = Select(t=w404, s="Scan axis 2", f=w408) -> (s? t:f=w414:dbl)
                  n239 = Select(t=w407, s="Scan axis 2", f=w404) -> (s? t:f=w413:dbl)
                  n240 = local read "Y RF Frequency Limits (MHz)"() -> (w409:T16)
                  n241 = local read "X RF Frequency Limits (MHz)"() -> (w410:T16)
                  n242 = local read "BD 1 Frequency 3 (MHz)"() -> (w417:dbl)
                  n243 = local read "BD 2 Frequency 2 (MHz)"() -> (w416:dbl)
                  n244 = local read "BD 2 Frequency 3 (MHz)"() -> (w415:dbl)
                  n245 = call "set RF board frequency - interlace.vi"("Board 2 Frequency Limits"=w409, "Board 1 Frequency Limits"=w410, "FPGA VI Reference In"=w402, "Board 2 Frequency 3 (MHz)"=w415, "Board 1 Frequency 3 (MHz)"=w417, "Board 2 Frequency 2 (MHz)"=w416, "Board 2 Frequency 1 (MHz)"=w413, "Board 1 Frequency 2 (MHz)"=w403, "Board 1 Frequency 1  (MHz)"=w414) -> ()  [unwired: 1 in, 2 out]
                }
                frame #1 {
                  n246 = And(x=w460, y=w457) -> (x .and. y?=w459:bool)
                  n247 = case "Only if were fishing and now formed tether" shown="False" w459 {
                    tunnel: w458 -> [w462 w477]
                    tunnel: [w461 w476] -> w456
                    tunnel: w455 -> [_ w472]
                    frame False {
                      n248 = local read "Fish for Tether"() -> (w461:bool)
                      n249 = case shown="False" w461 {
                        tunnel: w462 -> [w463 _]
                        frame False {
                          n250 = property on="BD 1 Frequency 1 (MHz)" class="DigNum (strict)"("Val(Sgnl)"=w463) -> ()  [unwired: 2 in, 2 out]
                        }
                        frame True {
                        }
                      }
                    }
                    frame True {
                      w476 = FALSE ("Fish for Tether")
                      n251 = call <vilib>:"Beep.vi"() -> ()  [unwired: 3 in, 9 out]
                      n252 = Number To Decimal String(number=w472, width (-)=i16 1) -> (decimal integer string=w470:string)
                      n253 = Concatenate Strings("Formed tether in ", w470, " attempt(s)." ("string")) -> (w467:string)
                      n254 = local read "Messages"() -> (w474:string)
                      n255 = local write "Fish for Tether"(w476) -> ()
                      n256 = call "Update messages.vi"("Message to add"=w467, "Old message string"=w474) -> ("New message string"=w473:string)
                      n257 = local write "Messages"(w473) -> ()
                      n258 = Get Date/Time In Seconds() -> (seconds since 1Jan1904=→"Time tether formed":timestamp)
                      n259 = local read "Flow ON during cal?"() -> (w464:bool)
                      n260 = property on="Sample Channel\nFlow" class="Bool (strict)"("Val(Sgnl)"=w464) -> (error out=w465:errorcluster)  [unwired: 2 in, 1 out]
                      n261 = case shown="\"2\", \"3\", \"4\", \"5\", \"6\"" "Then..." {
                        selector: "Then..." -> [_ w480]
                        tunnel: w477 -> [w479 _]
                        tunnel: w465 -> [_ _]
                        frame "1", Default {
                          n262 = property on="BD 1 Frequency 1 (MHz)" class="DigNum (strict)"("Val(Sgnl)"=w479) -> ()  [unwired: 2 in, 2 out]
                        }
                        frame "2", "3", "4", "5", "6" {
                          n263 = flat-sequence {
                            tunnel: w480 -> [w482]
                            frame #0 {
                              n264 = property on="Trap Delta (MHz)" class="DigNum (strict)"("Val(Sgnl)"="Move to Delta 1 (MHz)") -> ()  [unwired: 2 in, 2 out]
                            }
                            frame #1 {
                              n265 = case shown="\"5\", \"6\"" w482 {
                                selector: w482 -> [w485 w495 _]
                                frame "3", "4" {
                                n266 = flat-sequence {
                                tunnel: w485 -> [w486]
                                tunnel: [w486] -> w483
                                tunnel: [w488] -> w484
                                tunnel: w483 -> [w488]
                                tunnel: w484 -> [w492]
                                frame #0 {
                                n267 = property on="Green Laser ON" class="Bool (strict)"("Val(Sgnl)"=TRUE ("Value (Signaling)")) -> ()  [unwired: 2 in, 2 out]
                                }
                                frame #1 {
                                n268 = Multiply(x="Wait Before Save (s)", y=u32 1000 ("x")) -> (x*y=w490:u32)
                                n269 = Wait (ms)(milliseconds to wait=w490) -> ()  [unwired: 1 out]
                                }
                                frame #2 {
                                n270 = property on="Start Saving" class="Bool (strict)"("Value"=TRUE ("Start Saving")) -> ()  [unwired: 2 in, 2 out]
                                n271 = case shown="\"4\"" w492 {
                                frame Default {
                                }
                                frame "4" {
                                n272 = property on="Fl. Triggered..." class="Bool (strict)"("Val(Sgnl)"=TRUE ("Value (Signaling)")) -> ()  [unwired: 2 in, 2 out]
                                }
                                }
                                }
                                }
                                }
                                frame "5", "6" {
                                n273 = stacked-sequence {
                                tunnel: w495 -> [_ _ _ _ _ _ w507]
                                frame #0 {
                                n274 = Replace Array Subset(array=u32[] [0] ("Index Values"), new element="Raster Set Upon Tether", index=0) -> (w496:u32[])
                                n275 = property on="Saved AOD Raster Scan Parameter Sets" class="Arr (strict)"("Index Values"=w496) -> ()  [unwired: 2 in, 2 out]
                                }
                                frame #1 {
                                n276 = Wait (ms)(milliseconds to wait=u32 500) -> ()  [unwired: 1 out]
                                }
                                frame #2 {
                                n277 = property on="Load parameters" class="Bool (strict)"("Val(Sgnl)"=TRUE ("Value (Signaling)")) -> ()  [unwired: 2 in, 2 out]
                                n278 = case shown="True" "Green ON During Raster" {
                                frame False {
                                }
                                frame True {
                                n279 = property on="Green Laser ON" class="Bool (strict)"("Val(Sgnl)"=TRUE ("Value (Signaling)")) -> ()  [unwired: 2 in, 2 out]
                                }
                                }
                                }
                                frame #3 {
                                n280 = Wait (ms)(milliseconds to wait=u32 500) -> ()  [unwired: 1 out]
                                }
                                frame #4 {
                                n281 = property on="Trap Raster Scan" class="Bool (strict)"("Val(Sgnl)"=TRUE ("Value (Signaling)")) -> ()  [unwired: 2 in, 2 out]
                                }
                                frame #5 {
                                n282 = Wait (ms)(milliseconds to wait=u32 2000) -> ()  [unwired: 1 out]
                                }
                                frame #6 {
                                n283 = flat-sequence {
                                tunnel: w507 -> [w514]
                                frame #0 {
                                n284 = while {
                                stop <- w510 stop-if-true
                                n285 = local read "Raster Scanning..."() -> (w509:bool)
                                n286 = local read "Saving..."() -> (w512:bool)
                                n287 = Wait (ms)(milliseconds to wait=u32 100) -> ()  [unwired: 1 out]
                                n288 = Not(x=w512) -> (.not. x?=w511:bool)
                                n289 = Not(x=w509) -> (.not. x?=w508:bool)
                                n290 = And(x=w511, y=w508) -> (x .and. y?=w510:bool)
                                }
                                }
                                frame #1 {
                                n291 = local read "Tether"() -> (w515:bool)
                                n292 = case shown="True" w515 {
                                tunnel: w514 -> [_ w517]
                                frame False {
                                n293 = property on="Fish for Tether" class="Bool (strict)"("Val(Sgnl)"="Fish again after \nraster break?") -> ()  [unwired: 2 in, 2 out]
                                }
                                frame True {
                                n294 = stacked-sequence {
                                tunnel: w517 -> [_ w521 _ _]
                                frame #0 {
                                n295 = property on="Trap Delta (MHz)" class="DigNum (strict)"("Val(Sgnl)"="Move to Delta 2 (MHz)") -> ()  [unwired: 2 in, 2 out]
                                n296 = case shown="True" "Flow ON after\ntether testing?" {
                                frame False {
                                }
                                frame True {
                                n297 = property on="Sample Channel\nFlow" class="Bool (strict)"("Val(Sgnl)"=TRUE ("Value (Signaling)")) -> ()  [unwired: 2 in, 2 out]
                                }
                                }
                                }
                                frame #1 {
                                n298 = flat-sequence {
                                tunnel: w521 -> [w523]
                                frame #0 {
                                n299 = Wait (ms)(milliseconds to wait=u32 500) -> ()  [unwired: 1 out]
                                }
                                frame #1 {
                                n300 = case shown="\"6\"" w523 {
                                frame Default {
                                }
                                frame "6" {
                                n301 = property on="Green Laser ON" class="Bool (strict)"("Val(Sgnl)"=TRUE ("Green Laser ON/Interlacing")) -> ()  [unwired: 2 in, 2 out]
                                }
                                }
                                }
                                frame #2 {
                                n302 = Wait (ms)(milliseconds to wait=u32 500) -> ()  [unwired: 1 out]
                                }
                                frame #3 {
                                n303 = local write "Start Saving"("Save at end (5, 6)") -> ()
                                }
                                }
                                }
                                frame #2 {
                                n304 = local read "Bead Sep. Int. Time (s)"() -> (w529:dbl)
                                n305 = Multiply(x=w529, y=1000.0) -> (x*y=w528:dbl)
                                n306 = Wait (ms)(milliseconds to wait=w528) -> ()  [unwired: 1 out]
                                }
                                frame #3 {
                                n307 = property on="Remove Offset" class="Bool (strict)"("Val(Sgnl)"=TRUE ("Value (Signaling)")) -> ()  [unwired: 2 in, 2 out]
                                }
                                }
                                }
                                }
                                }
                                }
                                }
                                }
                                }
                                frame "2", Default {
                                }
                              }
                            }
                          }
                        }
                      }
                      "Tether" <- "Tether Alarm?"
                    }
                  }
                }
                frame #2 {
                  n308 = local read "Oscillate Set 1"() -> (w536:bool)
                  n309 = local read "Stop All"() -> (w534:bool)
                  n310 = Or(x=w536, y=w531) -> (x .or. y?=w533:bool)
                  n311 = Not(x=w533) -> (.not. x?=w535:bool)
                  n312 = Compound Arithmetic op=OR(w534, w535) -> (w532:bool)
                }
              }
              n313 = node-c288() -> ()  [unwired: 2 out]
            }
            n314 = node-c288(w377) -> ()  [unwired: 1 out]
          }
        }
      }
      event "Fl. Triggered...": Value Change {
        n315 = event-data() -> ()  [unwired: 7 out]
        n316 = case shown="True" "Fl. Triggered..." {
          frame False {
          }
          frame True {
            n317 = node-c288() -> (w547:T22)  [unwired: 4 out]
            n318 = timed-loop {
              timing: w547 -> [_]
              timing-out: [_] -> w546
              tunnel: "Action" -> [w555]
              shift-right: [w552] -> _
              shift-left: u8 255 -> [w554]
              shift-right: [w549] -> _
              shift-left: 255 -> [w551]
              stop <- w548 stop-if-true
              # "Reset confocal spot"
              n319 = node-c288() -> ()  [unwired: 2 out]
              n320 = flat-sequence {
                tunnel: w555 -> [w575]
                tunnel: w554 -> [w574]
                tunnel: [w573] -> w553
                tunnel: w551 -> [w560]
                tunnel: [w559] -> w550
                tunnel: [w954] -> w548
                tunnel: w553 -> [w953]
                tunnel: [w953] -> w552
                tunnel: [w952] -> w549
                tunnel: w550 -> [w952]
                frame #0 {
                  n321 = local read "Delta Fl. 2"() -> (w572:dbl)
                  n322 = local read "Delta Fl. 1"() -> (w567:dbl)
                  n323 = Multiply(x="Fl. Delta Thresh. (kHz)", y=1000.0) -> (x*y=w562:dbl)
                  n324 = Select(t=w567, s="APD to Watch", f=w572) -> (s? t:f=w563:dbl)
                  n325 = Greater?(x=w563, y=w562) -> (0:w568:bool)
                  n326 = Or(x="Force Yank", y=w568) -> (x .or. y?=w566:bool)
                  n327 = And(x=w566, y="Yank when?") -> (x .and. y?=w564:bool)
                  n328 = case shown="False" w564 {
                    tunnel: w575 -> [w578 w779]
                    tunnel: w574 -> [w580 w775]
                    tunnel: [w580 w773] -> w573
                    tunnel: w563 -> [w586 _]
                    tunnel: w562 -> [w585 _]
                    tunnel: "Force Yank" -> [w583 _]
                    tunnel: w560 -> [w582 w772]
                    tunnel: [w581 w772] -> w559
                    frame False {
                      n329 = Negate(x=w585) -> (-x=w577:dbl)
                      n330 = local write "Fl. High"(TRUE ("Fl. High")) -> ()
                      n331 = Less?(x=w586, y=w577) -> (x < y?=w584:bool)
                      n332 = Or(x=w583, y=w584) -> (x .or. y?=w579:bool)
                      n333 = case shown="True" w579 {
                        tunnel: w582 -> [w587 w597]
                        tunnel: [w587 w596] -> w581
                        tunnel: w578 -> [_ w595]
                        frame False {
                        }
                        frame True {
                          n334 = flat-sequence {
                            tunnel: w597 -> [w603]
                            tunnel: w595 -> [w600]
                            tunnel: [w602] -> w594
                            tunnel: [w601] -> w593
                            tunnel: [w600] -> w592
                            tunnel: w591 -> [w599]
                            tunnel: [w599] -> w590
                            tunnel: w589 -> [w598]
                            tunnel: [w598] -> w588
                            tunnel: [w674] -> w596
                            tunnel: w594 -> [w674]
                            tunnel: w593 -> [w673]
                            tunnel: w592 -> [w672]
                            tunnel: w590 -> [w671]
                            tunnel: w588 -> [w670]
                            frame #0 {
                              n335 = call <vilib>:"Beep.vi"() -> ()  [unwired: 12 in]
                              n336 = local write "Waiting"(FALSE ("Waiting")) -> ()
                              n337 = Increment(x=w603) -> (x+1=w602:i32)
                              n338 = case shown="\"Image\"" w600 {
                                tunnel: w602 -> [_ w608 _]
                                frame "Alarm", Default {
                                }
                                frame "Yank" {
                                n339 = flat-sequence {
                                tunnel: w608 -> [w611]
                                tunnel: [w610] -> w607
                                tunnel: [w609] -> w606
                                tunnel: w607 -> [w621]
                                tunnel: w606 -> [w622]
                                frame #0 {
                                n340 = local read "Yank Delay (s)"() -> (w614:dbl)
                                n341 = local read "N Array El"() -> (w609:u8)
                                n342 = Quotient & Remainder(x=w611, y=w609) -> (x-y*floor(x/y)=w610:i32)  [unwired: 1 out]
                                n343 = Multiply(x=w614, y=1000.0) -> (x*y=w612:dbl)
                                n344 = Wait (ms)(milliseconds to wait=w612) -> ()  [unwired: 1 out]
                                }
                                frame #1 {
                                n345 = local read "Yank to which?"() -> (w616:bool)
                                n346 = local read "Random Choice"() -> (w626:bool)
                                n347 = local read "Yank to Trap Delta (MHz)"() -> (w619:dbl[])
                                n348 = local read "Yank to SP"() -> (w620:dbl[])
                                n349 = Random Number (0-1)() -> (number: 0 to 1=w625:dbl)
                                n350 = Multiply(x=w622, y=w625) -> (x*y=w624:dbl)
                                n351 = Round Toward -Infinity(1:w624) -> (0:w623:dbl)
                                n352 = Select(t=w623, s=w626, f=w621) -> (s? t:f=w617:dbl)
                                n353 = Select(t=w619, s=w616, f=w620) -> (s? t:f=w618:dbl[])
                                n354 = Index Array(array=w618, index=w617) -> (element=w615:dbl)
                                n355 = case shown="True" w616 {
                                tunnel: w615 -> [w627 w654]
                                frame False {
                                n356 = flat-sequence {